vi "UHR-Fleezers Control (host) - 12.2.vi"() -> ()   [LabVIEW 2014] (continued)
        n1769 = local write "Saved Stage Positions"(w2524) -> ()
      }
      event "Move to Position": Value Change {
        n1770 = event-data() -> ()  [unwired: 1 in, 5 out]
        n1771 = flat-sequence {
          tunnel: w2531 -> [w2540]
          tunnel: w2530 -> [w2539]
          tunnel: [w2533] -> w2529
          tunnel: w2529 -> [w2550]
          frame #0 {
            # "Only change move time when saving move is T and calibrating is F"
            n1772 = local read "Saved Stage Positions"() -> (w2541:dbl[][])
            n1773 = property on="Saving Move" class="Bool (strict)"() -> ("Value"=w2534:bool)  [unwired: 2 in, 2 out]
            n1774 = property on="Calibrating..." class="Bool (strict)"() -> ("Value"=w2537:bool)  [unwired: 2 in, 2 out]
            n1775 = local read "Position"() -> (w2533:dbl)
            n1776 = call <vilib>:"Beep.vi"() -> ()  [unwired: 3 in, 9 out]
            n1777 = Not(x=w2537) -> (.not. x?=w2535:bool)
            n1778 = And(x=w2534, y=w2535) -> (x .and. y?=w2536:bool)
            n1779 = local write "Stage Moving"(TRUE ("Stage Moving")) -> ()
            n1780 = case shown="True" w2536 {
              frame False {
              }
              frame True {
                n1781 = Get Date/Time In Seconds() -> (seconds since 1Jan1904=w2549:timestamp)
                n1782 = Format Date/Time String(time format string (%c)="%H:%M:%S%3u", seconds (now)=w2549, UTC format=TRUE) -> (date/time string=w2546:string)
                n1783 = call <vilib>:"Space Constant.vi"() -> ("String"=w2545:string)
                n1784 = Concatenate Strings(w2546, w2545, "moving") -> (w2543:string)
                n1785 = property on="Move Time" class="Str"("Val(Sgnl)"=w2543) -> ()  [unwired: 2 in, 2 out]
              }
            }
            n1786 = call "move to saved stage position.vi"("error in"=w2539, "Stage VISA resource name in"=w2540, "Position"=w2533, "Saved Stage Positions"=w2541) -> ("error out"=w2538:errorcluster)  [unwired: 1 out]
            n1787 = local write "Stage Control Serial Error"(w2538) -> ()
          }
          frame #1 {
            n1788 = call <vilib>:"Beep.vi"() -> ()  [unwired: 3 in, 9 out]
            n1789 = property on="Saving Move" class="Bool (strict)"() -> ("Value"=w2554:bool)  [unwired: 2 in, 2 out]
            n1790 = local write "Stage Moving"(FALSE ("Stage Moving")) -> ()
            n1791 = property on="Calibrating..." class="Bool (strict)"() -> ("Value"=w2551:bool)  [unwired: 2 in, 2 out]
            n1792 = Not(x=w2551) -> (.not. x?=w2553:bool)
            n1793 = And(x=w2554, y=w2553) -> (x .and. y?=w2552:bool)
            n1794 = case shown="True" w2552 {
              tunnel: w2550 -> [_ w2556]
              frame False {
              }
              frame True {
                n1795 = Get Date/Time In Seconds() -> (seconds since 1Jan1904=w2564:timestamp)
                n1796 = Format Date/Time String(time format string (%c)="%H:%M:%S%3u", seconds (now)=w2564, UTC format=TRUE) -> (date/time string=w2561:string)
                n1797 = Number To Decimal String(number=w2556, width (-)=1) -> (decimal integer string=w2557:string)
                n1798 = call <vilib>:"Space Constant.vi"() -> ("String"=w2560:string)
                n1799 = Concatenate Strings(w2561, w2560, w2557) -> (w2559:string)
                n1800 = property on="Move Time" class="Str"("Val(Sgnl)"=w2559) -> ()  [unwired: 2 in, 2 out]
              }
            }
          }
        }
      }
      event "Move Cap. 1 (DNA Bottom)": Value Change {
        n1801 = event-data() -> ()  [unwired: 1 in, 5 out]
        n1802 = local write "Move Cap. 1 (DNA Bottom)"(FALSE ("Move Cap. 1 (DNA Right)")) -> ()
        n1803 = flat-sequence {
          tunnel: w2568 -> [w2571]
          tunnel: w2569 -> [w2572]
          tunnel: [w2572] -> w2566
          tunnel: [w2571] -> w2565
          tunnel: w2566 -> [w2574]
          tunnel: w2565 -> [w2573]
          frame #0 {
            n1804 = property on="Sample Channel\nFlow" class="Bool (strict)"("Val(Sgnl)"="Cap 1 Samp Flow ON") -> ()  [unwired: 2 in, 2 out]
          }
          frame #1 {
            n1805 = local read "Saved Stage Positions"() -> (w2584:dbl[][])
            n1806 = local write "Stage Moving"(TRUE ("Stage Moving")) -> ()
            n1807 = Array Subset(array=w2584, index (row)=0 ("index"), length (row)=1 ("length"), index (col)=1 ("index"), length (col)=3 ("length")) -> (w2581:dbl[][])
            n1808 = Reshape Array(w2581, 3 ("dimension size")) -> (w2579:dbl[])
            n1809 = Array To Cluster(array=w2579) -> (cluster=w2578:cluster{"[0]":dbl, "[1]":dbl, "[2]":dbl})
            n1810 = call "Set Stage Position.vi"("Position"=w2578, "error in"=w2573, "VISA resource name in"=w2574) -> ("error out"=w2577:errorcluster)  [unwired: 2 out]
            n1811 = local write "Stage Control Serial Error"(w2577) -> ()
          }
          frame #2 {
            n1812 = local write "Stage Moving"(FALSE ("Stage Moving")) -> ()
            n1813 = case shown="True" "Cap 1 Flow ON" {
              frame False {
              }
              frame True {
                n1814 = property on="Inject Pump 1" class="Bool (strict)"("Val(Sgnl)"=TRUE ("Value (Signaling)")) -> ()  [unwired: 2 in, 2 out]
              }
            }
            n1815 = call <vilib>:"Beep.vi"() -> ()  [unwired: 3 in, 9 out]
          }
          frame #3 {
            n1816 = property on="Sample Channel\nFlow" class="Bool (strict)"("Val(Sgnl)"=FALSE ("Value (Signaling)")) -> ()  [unwired: 2 in, 2 out]
            n1817 = local read "Cap. 2 BD T1?\n(ADig T1, DNA T2)"() -> (w2591:bool)
            n1818 = case shown="True" w2591 {
              tunnel: "Cap 1 T ON" -> [w2593 w2594]
              frame False {
                n1819 = property on="Trap 1 (ON/OFF)" class="Bool (strict)"("Val(Sgnl)"=w2593) -> ()  [unwired: 2 in, 2 out]
              }
              frame True {
                n1820 = property on="Trap 2 (ON/OFF)" class="Bool (strict)"("Val(Sgnl)"=w2594) -> ()  [unwired: 2 in, 2 out]
              }
            }
            n1821 = property on="Got DNA bead" class="Bool (strict)"("Key Focus"=TRUE) -> ()  [unwired: 2 in, 2 out]
          }
        }
      }
      event "Move Cap. 2 (ADig Top)": Value Change {
        n1822 = event-data() -> ()  [unwired: 1 in, 5 out]
        n1823 = local write "Move Cap. 2 (ADig Top)"(FALSE ("Move Cap. 2 (ADig Left)")) -> ()
        n1824 = flat-sequence {
          tunnel: w2598 -> [w2601]
          tunnel: w2599 -> [w2602]
          tunnel: [w2602] -> w2596
          tunnel: [w2601] -> w2595
          tunnel: w2596 -> [w2604]
          tunnel: w2595 -> [w2603]
          frame #0 {
            n1825 = property on="Sample Channel\nFlow" class="Bool (strict)"("Val(Sgnl)"="Cap 2 Samp Flow ON") -> ()  [unwired: 2 in, 2 out]
          }
          frame #1 {
            n1826 = local read "Saved Stage Positions"() -> (w2614:dbl[][])
            n1827 = local write "Stage Moving"(TRUE ("Stage Moving")) -> ()
            n1828 = Array Subset(array=w2614, index (row)=1 ("index"), length (row)=1 ("length"), index (col)=1 ("index"), length (col)=3 ("length")) -> (w2611:dbl[][])
            n1829 = disable-structure shown="Disabled" {
              frame Disabled {
                w2616 = FALSE ("Value (Signaling)")
                n1830 = property on="Trap 1 (ON/OFF)" class="Bool (strict)"("Val(Sgnl)"=w2616) -> ()  [unwired: 2 in, 2 out]
                n1831 = property on="Trap 1 (ON/OFF)" class="Bool (strict)"("Val(Sgnl)"=w2616) -> ()  [unwired: 2 in, 2 out]
              }
              frame Enabled {
              }
            }
            n1832 = Reshape Array(w2611, 3 ("dimension size")) -> (w2609:dbl[])
            n1833 = Array To Cluster(array=w2609) -> (cluster=w2608:cluster{"[0]":dbl, "[1]":dbl, "[2]":dbl})
            n1834 = call "Set Stage Position.vi"("Position"=w2608, "error in"=w2603, "VISA resource name in"=w2604) -> ("error out"=w2607:errorcluster)  [unwired: 2 out]
            n1835 = local write "Stage Control Serial Error"(w2607) -> ()
          }
          frame #2 {
            n1836 = local write "Stage Moving"(FALSE ("Stage Moving")) -> ()
            n1837 = call <vilib>:"Beep.vi"() -> ()  [unwired: 3 in, 9 out]
            n1838 = case shown="True" "Cap 2 Flow ON" {
              frame False {
              }
              frame True {
                n1839 = property on="Inject Pump 3" class="Bool (strict)"("Val(Sgnl)"=TRUE ("Value (Signaling)")) -> ()  [unwired: 2 in, 2 out]
              }
            }
          }
          frame #3 {
            n1840 = Wait (ms)(milliseconds to wait=u32 500) -> ()  [unwired: 1 out]
          }
          frame #4 {
            n1841 = local read "Cal @ (MHz)"() -> (w2622:dbl)
            n1842 = property on="Sample Channel\nFlow" class="Bool (strict)"("Val(Sgnl)"=FALSE ("Value (Signaling)")) -> ()  [unwired: 2 in, 2 out]
            n1843 = case shown="False" "Cap. 2 BD T1?\n(ADig T1, DNA T2)" {
              tunnel: "Cap 2 T ON" -> [w2627 w2628]
              frame False {
                n1844 = property on="Trap 2 (ON/OFF)" class="Bool (strict)"("Val(Sgnl)"=w2627) -> ()  [unwired: 2 in, 2 out]
              }
              frame True {
                n1845 = property on="Trap 1 (ON/OFF)" class="Bool (strict)"("Val(Sgnl)"=w2628) -> ()  [unwired: 2 in, 2 out]
              }
            }
            n1846 = property on="Got ADig bead" class="Bool (strict)"("Key Focus"=TRUE) -> ()  [unwired: 2 in, 2 out]
            n1847 = local write "Target"("Target\nON?") -> ()
            n1848 = property on="Trap D (MHz)" class="DigNum (strict)"("Val(Sgnl)"=w2622) -> ()  [unwired: 2 in, 2 out]
          }
        }
      }
      event "Read Harvard": Value Change {
        n1849 = event-data() -> ()  [unwired: 1 in, 5 out]
        n1850 = Concatenate Strings("write buffer", "\r") -> (w2633:string)
        n1851 = VISA Write(VISA resource name=w2631, write buffer=w2633, error in (no error)=w2630) -> (VISA resource name out=w2642:refnum<visa-resource-name>, error out=w2641:errorcluster)  [unwired: 1 out]
        n1852 = stacked-sequence {
          tunnel: [w2645] -> w2640
          tunnel: w2642 -> [w2645]
          tunnel: w2641 -> [w2644]
          tunnel: [w2644] -> w2635
          frame #0 {
            n1853 = Wait (ms)(milliseconds to wait=50) -> ()  [unwired: 1 out]
          }
        }
        n1854 = property class="Instr"(reference=w2640, error in=w2635) -> (reference out=w2639:refnum<visa-resource-name>, error out=w2637:errorcluster, "Serial Settings:Number of Bytes at Serial Port"=w2638:u32)
        "Serial Settings:Number of Bytes at Serial Port" <- w2638
        n1855 = VISA Read(VISA resource name=w2639, byte count=w2638, error in (no error)=w2637) -> (read buffer=w2636:string)  [unwired: 3 out]
        "read buffer" <- w2636
        n1856 = Fract/Exp String To Number(string=w2636) -> ()  [unwired: 5 out]
      }
      event "+z", "-z": Value Change {
        n1857 = event-data() -> ()  [unwired: 1 in, 5 out]
        n1858 = flat-sequence {
          tunnel: w2646 -> [w2668]
          tunnel: w2647 -> [w2648]
          frame #0 {
            n1859 = call "Read Stage Position.vi"("error in"=w2668, "VISA resource name in"=w2648) -> ("Current Position"=w2653:cluster{dbl, dbl, dbl}, "error out"=w2666:errorcluster, "VISA resource name out"=w2667:refnum<visa-resource-name>)  [unwired: 1 out]
            n1860 = local read "Saved Stage Positions"() -> (w2677:dbl[][])
            n1861 = Divide(x="z nudge increment (um)", y=1000.0) -> (x/y=w2665:dbl)
            n1862 = Boolean To (0,1)(Boolean="+z") -> (0, 1=w2657:i16)
            n1863 = Boolean To (0,1)(Boolean="-z") -> (0, 1=w2658:i16)
            n1864 = Array Subset(array=w2677, index (row)=1 ("index"), length (row)=1 ("length"), index (col)=1 ("index"), length (col)=3 ("length")) -> (w2674:dbl[][])
            n1865 = Multiply(x=w2657, y=w2665) -> (x*y=w2661:dbl)
            n1866 = Multiply(x=w2658, y=w2665) -> (x*y=w2659:dbl)
            n1867 = Unbundle(w2653) -> (w2651:dbl, w2650:dbl, w2654:dbl)
            n1868 = Negate(x=w2659) -> (-x=w2660:dbl)
            n1869 = Reshape Array(w2674, 3 ("dimension size")) -> (w2672:dbl[])
            n1870 = Add(x=w2661, y=w2660) -> (x+y=w2662:dbl)
            n1871 = Array To Cluster(array=w2672) -> ()  [unwired: 1 out]
            n1872 = Add(x=w2662, y=w2654) -> (x+y=w2652:dbl)
            n1873 = Bundle(cluster=w2653, w2651, w2650, w2652) -> (w2649:cluster{dbl, dbl, dbl})
            n1874 = call "Set Stage Position.vi"("Position"=w2649, "error in"=w2666, "VISA resource name in"=w2667) -> ("error out"=w2671:errorcluster)  [unwired: 2 out]
            n1875 = local write "Stage Moving"(TRUE ("Stage Moving")) -> ()
            n1876 = local write "Stage Control Serial Error"(w2671) -> ()
          }
          frame #1 {
            n1877 = local write "Stage Moving"(FALSE ("Stage Moving")) -> ()
            n1878 = call <vilib>:"Beep.vi"() -> ()  [unwired: 3 in, 9 out]
          }
        }
      }
      event "Cal/Data Acq. Spot": Value Change {
        n1879 = event-data() -> ()  [unwired: 1 in, 5 out]
        n1880 = flat-sequence {
          tunnel: w2686 -> [w2690]
          tunnel: w2687 -> [w2691]
          tunnel: [w2691] -> w2683
          tunnel: [w2690] -> w2682
          tunnel: w2683 -> [w2696]
          tunnel: w2682 -> [w2695]
          tunnel: ["Cal @ (MHz)"] -> w2680
          tunnel: [w2700] -> w2684
          tunnel: w2680 -> [w2700]
          tunnel: w2684 -> [w2711]
          tunnel: ["W/ Offset 1"] -> w2681
          tunnel: w2684 -> [w2732]
          tunnel: w2681 -> [w2730]
          frame #0 {
            n1881 = property on="Sample Channel\nFlow" class="Bool (strict)"("Val(Sgnl)"="Daq spot flow on") -> ()  [unwired: 2 in, 2 out]
            n1882 = Wait (ms)(milliseconds to wait=u32 250) -> ()  [unwired: 1 out]
          }
          frame #1 {
            n1883 = local read "Saved Stage Positions"() -> (w2693:dbl[][])
            n1884 = property on="Trap D (MHz)" class="DigNum (strict)"("Val(Sgnl)"="Cal @ (MHz)") -> ()  [unwired: 2 in, 2 out]
            n1885 = local write "Stage Moving"(TRUE ("Stage Moving")) -> ()
            n1886 = call "move to saved stage position.vi"("error in"=w2695, "Stage VISA resource name in"=w2696, "Position"="Cal Stage Position", "Saved Stage Positions"=w2693) -> ("error out"=w2694:errorcluster)  [unwired: 1 out]
            n1887 = local write "Stage Control Serial Error"(w2694) -> ()
          }
          frame #2 {
            n1888 = local write "Stage Moving"(FALSE ("Stage Moving")) -> ()
            n1889 = property on="Sample Channel\nFlow" class="Bool (strict)"("Val(Sgnl)"="Flow ON\nduring cal?") -> ()  [unwired: 2 in, 2 out]
            n1890 = call <vilib>:"Beep.vi"() -> ()  [unwired: 3 in, 9 out]
          }
          frame #3 {
            n1891 = local read "Wait Before Save (s)"() -> (w2703:u32)
            n1892 = Multiply(x=w2703, y=u32 1000 ("milliseconds to wait")) -> (x*y=w2704:u32)
            n1893 = Wait (ms)(milliseconds to wait=w2704) -> ()  [unwired: 1 out]
          }
          frame #4 {
            n1894 = property on="Save Calibration" class="Bool (strict)"("Val(Sgnl)"=TRUE ("Value (Signaling)")) -> ()  [unwired: 2 in, 2 out]
          }
          frame #5 {
            n1895 = Wait (ms)(milliseconds to wait=u32 2000) -> ()  [unwired: 1 out]
          }
          frame #6 {
            # "Check to see if \nsaving done"
            n1896 = while {
              stop <- w2707 stop-if-true
              n1897 = local read "Saving..."() -> (w2708:bool)
              n1898 = Wait (ms)(milliseconds to wait=u32 100) -> ()  [unwired: 1 out]
              n1899 = Not(x=w2708) -> (.not. x?=w2707:bool)
            }
          }
          frame #7 {
            n1900 = case shown="True" "W/ Offset 1" {
              tunnel: w2711 -> [_ w2712]
              frame False {
              }
              frame True {
                n1901 = stacked-sequence {
                  tunnel: w2712 -> [_ _ _ _ _ _ _ w2729]
                  frame #0 {
                    n1902 = property on="Trap D (MHz)" class="DigNum (strict)"("Val(Sgnl)"="Offset 1 Start (MHz)") -> ()  [unwired: 2 in, 2 out]
                    n1903 = Replace Array Subset(array=u32[] [0] ("Index Values"), new element="Offset 1 Set", index=0) -> (w2713:u32[])
                    n1904 = property on="Saved AOD Raster Scan Parameter Sets" class="Arr (strict)"("Index Values"=w2713) -> ()  [unwired: 2 in, 2 out]
                  }
                  frame #1 {
                    n1905 = Wait (ms)(milliseconds to wait=u32 200) -> ()  [unwired: 1 out]
                  }
                  frame #2 {
                    n1906 = property on="Load parameters" class="Bool (strict)"("Val(Sgnl)"=TRUE ("Value (Signaling)")) -> ()  [unwired: 2 in, 2 out]
                  }
                  frame #3 {
                    n1907 = Wait (ms)(milliseconds to wait=u32 200) -> ()  [unwired: 1 out]
                  }
                  frame #4 {
                    n1908 = property on="Trap Raster Scan" class="Bool (strict)"("Val(Sgnl)"=TRUE ("Value (Signaling)")) -> ()  [unwired: 2 in, 2 out]
                  }
                  frame #5 {
                    n1909 = Wait (ms)(milliseconds to wait=u32 2000) -> ()  [unwired: 1 out]
                  }
                  frame #6 {
                    n1910 = while {
                      stop <- w2726 stop-if-true
                      n1911 = local read "Raster Scanning..."() -> (w2728:bool)
                      n1912 = local read "Saving..."() -> (w2724:bool)
                      n1913 = Wait (ms)(milliseconds to wait=u32 100) -> ()  [unwired: 1 out]
                      n1914 = Not(x=w2724) -> (.not. x?=w2723:bool)
                      n1915 = Not(x=w2728) -> (.not. x?=w2725:bool)
                      n1916 = And(x=w2725, y=w2723) -> (x .and. y?=w2726:bool)
                    }
                  }
                  frame #7 {
                    n1917 = property on="Trap D (MHz)" class="DigNum (strict)"("Val(Sgnl)"=w2729) -> ()  [unwired: 2 in, 2 out]
                  }
                }
              }
            }
          }
          frame #8 {
            n1918 = local read "Save ave N"() -> (w2731:dbl)
            n1919 = case shown="False" "W/ Offset 2" {
              tunnel: w2732 -> [_ w2739]
              tunnel: w2731 -> [_ w2738]
              tunnel: w2730 -> [w2734 _]
              frame False {
                n1920 = case shown="False" w2734 {
                  frame False {
                    n1921 = Multiply(x="Cal read wait (s)", y=u32 1000 ("milliseconds to wait")) -> (x*y=w2736:u32)
                    n1922 = Wait (ms)(milliseconds to wait=w2736) -> ()  [unwired: 1 out]
                  }
                  frame True {
                  }
                }
              }
              frame True {
                n1923 = stacked-sequence {
                  tunnel: w2739 -> [_ _ _ _ _ _ _ _ _ w2760 _ _]
                  tunnel: w2738 -> [_ _ _ _ _ _ _ _ _ w2758 _ _]
                  frame #0 {
                    n1924 = property on="Save ave N" class="DigNum (strict)"("Val(Sgnl)"=1.0 ("Value (Signaling)")) -> ()  [unwired: 2 in, 2 out]
                  }
                  frame #1 {
                    n1925 = Wait (ms)(milliseconds to wait=u32 500) -> ()  [unwired: 1 out]
                  }
                  frame #2 {
                    n1926 = property on="Trap D (MHz)" class="DigNum (strict)"("Val(Sgnl)"="Offset 2 Start (MHz)") -> ()  [unwired: 2 in, 2 out]
                    n1927 = Replace Array Subset(array=u32[] [0] ("Index Values"), new element="Offset 2 Set", index=0) -> (w2744:u32[])
                    n1928 = property on="Saved AOD Raster Scan Parameter Sets" class="Arr (strict)"("Index Values"=w2744) -> ()  [unwired: 2 in, 2 out]
                  }
                  frame #3 {
                    n1929 = Wait (ms)(milliseconds to wait=u32 500) -> ()  [unwired: 1 out]
                  }
                  frame #4 {
                    n1930 = property on="Load parameters" class="Bool (strict)"("Val(Sgnl)"=TRUE ("Value (Signaling)")) -> ()  [unwired: 2 in, 2 out]
                  }
                  frame #5 {
                    n1931 = Wait (ms)(milliseconds to wait=u32 500) -> ()  [unwired: 1 out]
                  }
                  frame #6 {
                    n1932 = property on="Trap Raster Scan" class="Bool (strict)"("Val(Sgnl)"=TRUE ("Value (Signaling)")) -> ()  [unwired: 2 in, 2 out]
                  }
                  frame #7 {
                    n1933 = Wait (ms)(milliseconds to wait=u32 2000) -> ()  [unwired: 1 out]
                  }
                  frame #8 {
                    n1934 = while {
                      stop <- w2753 stop-if-true
                      n1935 = local read "Raster Scanning..."() -> (w2756:bool)
                      n1936 = local read "Saving..."() -> (w2754:bool)
                      n1937 = Wait (ms)(milliseconds to wait=u32 100) -> ()  [unwired: 1 out]
                      n1938 = Not(x=w2754) -> (.not. x?=w2752:bool)
                      n1939 = Not(x=w2756) -> (.not. x?=w2755:bool)
                      n1940 = And(x=w2755, y=w2752) -> (x .and. y?=w2753:bool)
                    }
                  }
                  frame #9 {
                    n1941 = property on="Trap D (MHz)" class="DigNum (strict)"("Val(Sgnl)"=w2760) -> ()  [unwired: 2 in, 2 out]
                    n1942 = property on="Saved AOD Raster Scan Parameter Sets" class="Arr (strict)"("Index Values"=u32[] [0]) -> ()  [unwired: 2 in, 2 out]
                    n1943 = property on="Save ave N" class="DigNum (strict)"("Val(Sgnl)"=w2758) -> ()  [unwired: 2 in, 2 out]
                  }
                  frame #10 {
                    n1944 = Wait (ms)(milliseconds to wait=u32 500) -> ()  [unwired: 1 out]
                  }
                  frame #11 {
                    n1945 = property on="Load parameters" class="Bool (strict)"("Val(Sgnl)"=TRUE ("Value (Signaling)")) -> ()  [unwired: 2 in, 2 out]
                  }
                }
              }
            }
          }
          frame #9 {
            n1946 = property on="Read Cal" class="Bool (strict)"("Val(Sgnl)"=TRUE ("Value (Signaling)")) -> ()  [unwired: 2 in, 2 out]
          }
          frame #10 {
            n1947 = Wait (ms)(milliseconds to wait=u32 1000) -> ()  [unwired: 1 out]
          }
          frame #11 {
            n1948 = property on="Fish" class="Bool (strict)"("Val(Sgnl)"=TRUE ("Value (Signaling)")) -> ()  [unwired: 2 in, 2 out]
          }
        }
        n1949 = local write "Cal/Data Acq. Spot"(FALSE ("Cal/Data Acq. Spot")) -> ()
      }
      event "Dump Beads": Value Change {
        n1950 = event-data() -> ()  [unwired: 1 in, 5 out]
        n1951 = flat-sequence {
          tunnel: ["Dump spot flow on?"] -> w2766
          tunnel: [w2778] -> w2767
          tunnel: w2766 -> [w2778]
          tunnel: w2770 -> [w2783]
          tunnel: w2769 -> [w2782]
          tunnel: [w2780] -> w2768
          tunnel: w2767 -> [w2780]
          tunnel: w2768 -> [w2794]
          frame #0 {
            w2771 = FALSE ("Value (Signaling)")
            n1952 = local read "Saving..."() -> (w2773:bool)
            n1953 = local write "Dump Beads"(FALSE ("Dump Beads")) -> ()
            n1954 = property on="Inject Pump 3" class="Bool (strict)"("Val(Sgnl)"=w2771) -> ()  [unwired: 2 in, 2 out]
            n1955 = property on="Inject Pump 1" class="Bool (strict)"("Val(Sgnl)"=w2771) -> ()  [unwired: 2 in, 2 out]
            n1956 = local write "Stop Saving"(w2773) -> ()
            n1957 = local write "Fish"(w2771) -> ()
          }
          frame #1 {
            w2774 = TRUE
            w2775 = FALSE ("Fl. Triggered...")
            n1958 = case shown="True" "Dump spot flow on?" {
              frame False {
              }
              frame True {
                n1959 = property on="Sample Channel\nFlow" class="Bool (strict)"("Val(Sgnl)"=TRUE ("Stage Moving")) -> ()  [unwired: 2 in, 2 out]
              }
            }
            n1960 = local write "Fl. Triggered..."(w2775) -> ()
            n1961 = local write "Tether"(w2775) -> ()
            n1962 = local write "Multiple tether"(w2775) -> ()
            n1963 = local write "Good tether"(w2775) -> ()
            n1964 = property on="Green ON/Interlacing" class="Bool (strict)"("Val(Sgnl)"=w2775) -> ()  [unwired: 2 in, 2 out]
            n1965 = property on="Trap Pos. FB ON" class="Bool (strict)"("Val(Sgnl)"=w2775) -> ()  [unwired: 2 in, 2 out]
            n1966 = property on="Trap Trig. Fl." class="Bool (strict)"("Val(Sgnl)"=w2775) -> ()  [unwired: 2 in, 2 out]
            n1967 = local write "Bad fit"(w2775) -> ()
            n1968 = local write "Hysteresis"(w2775) -> ()
            n1969 = property on="Fl. Triggered..." class="Bool (strict)"("Val(Sgnl)"=w2775) -> ()  [unwired: 2 in, 2 out]
            n1970 = local write "Restart DMA? (AOD)"(w2774) -> ()
            n1971 = local write "Save scans"(w2774) -> ()
            n1972 = property on="Dip for Protein" class="Bool (strict)"("Val(Sgnl)"=w2775) -> ()  [unwired: 2 in, 2 out]
            n1973 = property on="Pause dwell" class="Bool (strict)"("Val(Sgnl)"=w2775) -> ()  [unwired: 2 in, 2 out]
          }
          frame #2 {
            n1974 = property on="Trap Pos. FB Offset Factor" class="DigNum (strict)"("Val(Sgnl)"=i64 0 ("Value (Signaling)")) -> ()  [unwired: 2 in, 2 out]
          }
          frame #3 {
            n1975 = local read "Saved Stage Positions"() -> (w2784:dbl[][])
            n1976 = Array Subset(array=w2784, index (row)=3 ("index"), length (row)=1 ("length"), index (col)=1 ("index"), length (col)=3 ("length")) -> (w2789:dbl[][])
            n1977 = local write "Stage Moving"(TRUE ("Stage Moving")) -> ()
            n1978 = Reshape Array(w2789, 3 ("dimension size")) -> (w2787:dbl[])
            n1979 = Array To Cluster(array=w2787) -> (cluster=w2786:cluster{"[0]":dbl, "[1]":dbl, "[2]":dbl})
            n1980 = call "Set Stage Position.vi"("Position"=w2786, "error in"=w2782, "VISA resource name in"=w2783) -> ()  [unwired: 3 out]
          }
          frame #4 {
            w2795 = FALSE ("Value (Signaling)")
            n1981 = case shown="True" w2794 {
              frame False {
              }
              frame True {
                n1982 = property on="Sample Channel\nFlow" class="Bool (strict)"("Val(Sgnl)"=FALSE ("Stage Moving")) -> ()  [unwired: 2 in, 2 out]
              }
            }
            n1983 = property on="Trap 1 (ON/OFF)" class="Bool (strict)"("Val(Sgnl)"=w2795) -> ()  [unwired: 2 in, 2 out]
            n1984 = property on="Trap 2 (ON/OFF)" class="Bool (strict)"("Val(Sgnl)"=w2795) -> ()  [unwired: 2 in, 2 out]
            n1985 = call <vilib>:"Beep.vi"() -> ()  [unwired: 3 in, 9 out]
            n1986 = local write "Fish"(FALSE ("Fish for Tether")) -> ()
          }
          frame #5 {
            n1987 = property on="Move Cap. 2 (ADig Top)" class="Bool (strict)"("Val(Sgnl)"=TRUE ("Value (Signaling)")) -> ()  [unwired: 2 in, 2 out]
            n1988 = property on="Tab Control" class="TabCtl (strict)"("Val(Sgnl)"=T34."Status" ("Value (Signaling)")) -> ()  [unwired: 2 in, 2 out]
          }
        }
      }
      event "Dip for Protein": Value Change {
        n1989 = event-data() -> ()  [unwired: 1 in, 5 out]
        n1990 = local read "Calibrating..."() -> (w2802:bool)
        n1991 = local read "Saving Move"() -> (w2800:bool)
        n1992 = Not(x=w2802) -> (.not. x?=w2801:bool)
        n1993 = And(x=w2800, y=w2801) -> (x .and. y?=w2799:bool)
        n1994 = case shown="True" "Dip for Protein" {
          tunnel: w2805 -> [_ w2808]
          tunnel: w2804 -> [_ w2807]
          tunnel: w2799 -> [_ w2806]
          frame False {
          }
          frame True {
            n1995 = while {
              tunnel: w2808 -> [w2821]
              tunnel: w2807 -> [w2820]
              tunnel: w2806 -> [w2809]
              i -> [w2816]
              stop <- w2811 stop-if-true
              n1996 = Increment(x=w2816) -> (x+1=→"Dip #":i32)
              n1997 = flat-sequence {
                tunnel: w2820 -> [w2832]
                tunnel: w2821 -> [w2833]
                tunnel: [w2833] -> w2825
                tunnel: [w2832] -> w2824
                tunnel: [w2826] -> w2812
                tunnel: [w2840] -> w2819
                tunnel: [w2841] -> w2818
                tunnel: w2825 -> [w2842]
                tunnel: w2824 -> [w2843]
                tunnel: [w2838] -> w2813
                tunnel: w2812 -> [w2838]
                tunnel: w2809 -> [w2837]
                tunnel: ["Dip Stage \nPosition"] -> w2810
                tunnel: [w2860] -> w2823
                tunnel: w2819 -> [w2860]
                tunnel: [w2859] -> w2822
                tunnel: w2818 -> [w2859]
                tunnel: [w2856] -> w2817
                tunnel: [w2855] -> w2814
                tunnel: w2813 -> [w2855]
                tunnel: w2809 -> [w2854]
                tunnel: w2810 -> [w2853]
                tunnel: w2822 -> [w2892]
                tunnel: w2823 -> [w2893]
                tunnel: w2817 -> [w2894]
                tunnel: w2814 -> [w2891]
                tunnel: w2809 -> [w2890]
                tunnel: w2809 -> [w2889]
                tunnel: [w2977] -> w2811
                frame #0 {
                  n1998 = local read "Trap Pos. FB ON"() -> (w2826:bool)
                  n1999 = Compound Arithmetic op=AND("Flow ON\nduring dip?", "FB OFF when \nflow ON", w2826) -> (w2827:bool)
                  n2000 = case shown="True" "Move trap \nbefore dip move?" {
                    frame False {
                    }
                    frame True {
                      n2001 = property on="Trap D (MHz)" class="DigNum (strict)"("Val(Sgnl)"="Dipping D (MHz)") -> ()  [unwired: 2 in, 2 out]
                    }
                  }
                  n2002 = property on="Green ON/Interlacing" class="Bool (strict)"("Val(Sgnl)"="Green ON\nbefore dip?") -> ()  [unwired: 2 in, 2 out]
                  n2003 = property on="Sample Channel\nFlow" class="Bool (strict)"("Val(Sgnl)"="Flow ON\nduring dip?") -> ()  [unwired: 2 in, 2 out]
                  n2004 = case shown="True" w2827 {
                    frame False {
                    }
                    frame True {
                      n2005 = property on="Trap Pos. FB ON" class="Bool (strict)"("Val(Sgnl)"=FALSE ("Value (Signaling)")) -> ()  [unwired: 2 in, 2 out]
                    }
                  }
                }
                frame #1 {
                  n2006 = local read "Saved Stage Positions"() -> (w2844:dbl[][])
                  n2007 = local write "Cancel dwell"(FALSE ("Cancel dwell")) -> ()
                  n2008 = call "move to saved stage position.vi"("error in"=w2843, "Stage VISA resource name in"=w2842, "Position"="Dip Stage \nPosition", "Saved Stage Positions"=w2844) -> ("VISA resource name out"=w2840:refnum<visa-resource-name>, "error out"=w2841:errorcluster)
                  n2009 = case shown="True" w2837 {
                    frame False {
                    }
                    frame True {
                      n2010 = Get Date/Time In Seconds() -> (seconds since 1Jan1904=w2851:timestamp)
                      n2011 = call <vilib>:"Space Constant.vi"() -> ("String"=w2848:string)
                      n2012 = local write "Stage Moving"(TRUE) -> ()
                      n2013 = Format Date/Time String(time format string (%c)="%H:%M:%S%3u", seconds (now)=w2851, UTC format=TRUE) -> (date/time string=w2849:string)
                      n2014 = Concatenate Strings(w2849, w2848, "moving") -> (w2846:string)
                      n2015 = property on="Move Time" class="Str"("Val(Sgnl)"=w2846) -> ()  [unwired: 2 in, 2 out]
                    }
                  }
                }
                frame #2 {
                  n2016 = node-c288() -> (w2858:T26)  [unwired: 4 in]
                  n2017 = timed-loop {
                    timing: w2858 -> [_]
                    timing-out: [_] -> w2857
                    tunnel: [w2874] -> w2856
                    i -> [w2871]
                    stop <- w2875 stop-if-true
                    n2018 = node-c288() -> ()  [unwired: 1 in, 1 out]
                    n2019 = Greater Or Equal?(x=w2871, y="Dip Duration (s)") -> (x >= y?=w2883:bool)
                    n2020 = local read "Dip for Protein"() -> (w2876:bool)
                    n2021 = local read "Dump Beads"() -> (w2873:bool)
                    n2022 = local read "Cancel dwell"() -> (w2882:bool)
                    n2023 = local read "Pause dwell"() -> (w2879:bool)
                    n2024 = Not(x=w2876) -> (.not. x?=w2881:bool)
                    n2025 = Compound Arithmetic op=OR(w2882, w2883, w2881) -> (w2880:bool)
                    n2026 = Select(t=FALSE, s=w2879, f=w2880) -> (s? t:f=w2877:bool)
                    n2027 = Not(x=w2873) -> (.not. x?=w2872:bool)
                    n2028 = node-c288() -> ()  [unwired: 1 in, 1 out]
                    n2029 = And(x=w2876, y=w2872) -> (x .and. y?=w2874:bool)
                    n2030 = Or(x=w2877, y=w2873) -> (x .or. y?=w2875:bool)
                    "Dip Time (s)" <- w2871
                  }
                  n2031 = case shown="True" w2854 {
                    tunnel: w2853 -> [_ w2861]
                    frame False {
                    }
                    frame True {
                      n2032 = Get Date/Time In Seconds() -> (seconds since 1Jan1904=w2869:timestamp)
                      n2033 = call <vilib>:"Space Constant.vi"() -> ("String"=w2866:string)
                      n2034 = Number To Decimal String(number=w2861, width (-)=1) -> (decimal integer string=w2864:string)
                      n2035 = local write "Stage Moving"(FALSE) -> ()
                      n2036 = Format Date/Time String(time format string (%c)="%H:%M:%S%3u", seconds (now)=w2869, UTC format=TRUE) -> (date/time string=w2867:string)
                      n2037 = Concatenate Strings(w2867, w2866, w2864) -> (w2865:string)
                      n2038 = property on="Move Time" class="Str"("Val(Sgnl)"=w2865) -> ()  [unwired: 2 in, 2 out]
                    }
                  }
                  n2039 = node-c288(w2857) -> ()  [unwired: 1 out]
                }
                frame #3 {
                  n2040 = case shown="True" w2894 {
                    tunnel: w2893 -> [_ w2902]
                    tunnel: w2892 -> [_ w2901]
                    tunnel: w2891 -> [_ w2898]
                    tunnel: w2890 -> [_ w2897]
                    tunnel: w2889 -> [_ w2895]
                    frame False {
                    }
                    frame True {
                      n2041 = flat-sequence {
                        tunnel: w2901 -> [w2906]
                        tunnel: w2902 -> [w2907]
                        tunnel: [w2907] -> w2900
                        tunnel: [w2906] -> w2899
                        tunnel: w2898 -> [w2903]
                        tunnel: w2900 -> [w2919]
                        tunnel: w2899 -> [w2918]
                        tunnel: w2897 -> [w2915]
                        tunnel: ["Return Stage \nPosition"] -> w2896
                        tunnel: w2898 -> [w2937]
                        tunnel: w2896 -> [w2935]
                        tunnel: w2895 -> [w2934]
                        frame #0 {
                          n2042 = local read "Sample Channel\nFlow"() -> (w2905:bool)
                          n2043 = case shown="True" w2905 {
                            tunnel: "Flow ON \nduring return\nfrom dip?" -> [w2908 w2911]
                            tunnel: w2903 -> [_ w2910]
                            frame False {
                              n2044 = case shown="True" w2908 {
                                frame False {
                                }
                                frame True {
                                n2045 = property on="Sample Channel\nFlow" class="Bool (strict)"("Val(Sgnl)"=TRUE ("Value (Signaling)")) -> ()  [unwired: 2 in, 2 out]
                                }
                              }
                            }
                            frame True {
                              n2046 = case shown="False" w2911 {
                                tunnel: w2910 -> [w2912 _]
                                frame False {
                                n2047 = property on="Trap Pos. FB ON" class="Bool (strict)"("Val(Sgnl)"=w2912) -> ()  [unwired: 2 in, 2 out]
                                n2048 = property on="Sample Channel\nFlow" class="Bool (strict)"("Val(Sgnl)"=FALSE ("Value (Signaling)")) -> ()  [unwired: 2 in, 2 out]
                                }
                                frame True {
                                }
                              }
                            }
                          }
                        }
                        frame #1 {
                          # "For turning on green laser before stage reaches lower spot"
                          n2049 = case shown="True" "Green ON\nafter start\nreturn?" {
                            frame False {
                            }
                            frame True {
                              n2050 = flat-sequence {
                                frame #0 {
                                n2051 = Multiply(x="Green delay after \nstart return (s)", y=1000.0) -> (x*y=w2931:dbl)
                                n2052 = Wait (ms)(milliseconds to wait=w2931) -> ()  [unwired: 1 out]
                                }
                                frame #1 {
                                n2053 = property on="Green ON/Interlacing" class="Bool (strict)"("Val(Sgnl)"=TRUE ("Value (Signaling)")) -> ()  [unwired: 2 in, 2 out]
                                }
                              }
                            }
                          }
                          n2054 = local read "Saved Stage Positions"() -> (w2921:dbl[][])
                          n2055 = local write "Cancel dwell"(FALSE ("Cancel dwell")) -> ()
                          n2056 = call "move to saved stage position.vi"("error in"=w2918, "Stage VISA resource name in"=w2919, "Position"="Return Stage \nPosition", "Saved Stage Positions"=w2921) -> ("error out"=w2920:errorcluster)  [unwired: 1 out]
                          n2057 = local write "Stage Control Serial Error"(w2920) -> ()
                          n2058 = case shown="True" w2915 {
                            frame False {
                            }
                            frame True {
                              n2059 = Get Date/Time In Seconds() -> (seconds since 1Jan1904=w2928:timestamp)
                              n2060 = call <vilib>:"Space Constant.vi"() -> ("String"=w2925:string)
                              n2061 = local write "Stage Moving"(TRUE) -> ()
                              n2062 = Format Date/Time String(time format string (%c)="%H:%M:%S%3u", seconds (now)=w2928, UTC format=TRUE) -> (date/time string=w2926:string)
                              n2063 = Concatenate Strings(w2926, w2925, "moving") -> (w2923:string)
                              n2064 = property on="Move Time" class="Str"("Val(Sgnl)"=w2923) -> ()  [unwired: 2 in, 2 out]
                            }
                          }
                        }
                        frame #2 {
                          n2065 = case shown="True" w2934 {
                            tunnel: w2935 -> [_ w2941]
                            frame False {
                            }
                            frame True {
                              n2066 = Get Date/Time In Seconds() -> (seconds since 1Jan1904=w2949:timestamp)
                              n2067 = call <vilib>:"Space Constant.vi"() -> ("String"=w2946:string)
                              n2068 = Number To Decimal String(number=w2941, width (-)=1) -> (decimal integer string=w2944:string)
                              n2069 = local write "Stage Moving"(FALSE) -> ()
                              n2070 = Format Date/Time String(time format string (%c)="%H:%M:%S%3u", seconds (now)=w2949, UTC format=TRUE) -> (date/time string=w2947:string)
                              n2071 = Concatenate Strings(w2947, w2946, w2944) -> (w2945:string)
                              n2072 = property on="Move Time" class="Str"("Val(Sgnl)"=w2945) -> ()  [unwired: 2 in, 2 out]
                            }
                          }
                          n2073 = case shown="True" "Move trap after return?" {
                            frame False {
                            }
                            frame True {
                              n2074 = property on="Trap D (MHz)" class="DigNum (strict)"("Val(Sgnl)"="Dip Trap D 2 (MHz)") -> ()  [unwired: 2 in, 2 out]
                            }
                          }
                          n2075 = property on="Trap Pos. FB ON" class="Bool (strict)"("Val(Sgnl)"=w2937) -> ()  [unwired: 2 in, 2 out]
                          n2076 = case shown="True" "Green ON \nafter return?" {
                            frame False {
                            }
                            frame True {
                              n2077 = property on="Green ON/Interlacing" class="Bool (strict)"("Val(Sgnl)"=TRUE ("Value (Signaling)")) -> ()  [unwired: 2 in, 2 out]
                            }
                          }
                          n2078 = case shown="True" "Save data after return?" {
                            frame False {
                            }
                            frame True {
                              n2079 = property on="Start Saving" class="Bool (strict)"("Val(Sgnl)"=TRUE ("Value (Signaling)")) -> ()  [unwired: 2 in, 2 out]
                            }
                          }
                          n2080 = property on="Sample Channel\nFlow" class="Bool (strict)"("Val(Sgnl)"="Flow ON\nduring daq?") -> ()  [unwired: 2 in, 2 out]
                        }
                        frame #3 {
                          n2081 = node-c288() -> (w2955:T26)  [unwired: 4 in]
                          n2082 = timed-loop {
                            timing: w2955 -> [_]
                            timing-out: [_] -> w2954
                            i -> [w2956]
                            stop <- w2958 stop-if-true
                            n2083 = node-c288() -> ()  [unwired: 1 in, 1 out]
                            n2084 = local read "Dump Beads"() -> (w2957:bool)
                            n2085 = Greater Or Equal?(x=w2956, y="Dwell Duration (s)") -> (x >= y?=w2963:bool)
                            n2086 = local read "Dip for Protein"() -> (w2960:bool)
                            n2087 = Not(x=w2960) -> (.not. x?=w2959:bool)
                            n2088 = Compound Arithmetic op=OR(w2963, "Cancel dwell", w2959) -> (w2962:bool)
                            n2089 = node-c288() -> ()  [unwired: 1 in, 1 out]
                            n2090 = Select(t=FALSE, s="Pause dwell", f=w2962) -> (s? t:f=w2965:bool)
                            n2091 = Or(x=w2965, y=w2957) -> (x .or. y?=w2958:bool)
                            "Dwell Time (s)" <- w2956
                          }
                          n2092 = node-c288(w2954) -> ()  [unwired: 1 out]
                        }
                      }
                    }
                  }
                }
                frame #4 {
                  n2093 = local read "Dip for Protein"() -> (w2974:bool)
                  n2094 = local read "Tether"() -> (w2973:bool)
                  n2095 = local read "Dump Beads"() -> (w2975:bool)
                  n2096 = local write "Cancel dwell"(FALSE ("Cancel dwell")) -> ()
                  n2097 = Not(x=w2973) -> (.not. x?=w2972:bool)
                  n2098 = Not(x=w2974) -> (.not. x?=w2978:bool)
                  n2099 = Not(x="Cont. Repeat Dipping?") -> (.not. x?=w2980:bool)
                  n2100 = Compound Arithmetic op=OR(w2972, w2978, w2980, w2975) -> (w2977:bool)
                }
              }
            }
          }
        }
      }
      event "Profile": Value Change {
        n2101 = event-data() -> ()  [unwired: 1 in, 5 out]
        n2102 = flat-sequence {
          tunnel: w2989 -> [w2992]
          tunnel: w2988 -> [w3000]
          tunnel: [w2994] -> w2987
          tunnel: [w2993] -> w2986
          tunnel: [w2991] -> w2984
          tunnel: [w2990] -> w2981
          tunnel: w2987 -> [w3007]
          tunnel: w2986 -> [w3006]
          tunnel: [w3004] -> w2985
          tunnel: w2984 -> [w3005]
          tunnel: [w3003] -> w2983
          tunnel: [w3002] -> w2982
          tunnel: w2981 -> [w3002]
          tunnel: w2985 -> [w3011]
          tunnel: w2983 -> [w3010]
          tunnel: w2982 -> [w3009]
          frame #0 {
            n2103 = call "Read Stage Position.vi"("error in"=w3000, "VISA resource name in"=w2992) -> ("Current Position"=w2990:cluster{dbl, dbl, dbl}, "error out"=w2993:errorcluster, "VISA resource name out"=w2991:refnum<visa-resource-name>)  [unwired: 1 out]
            "Current Position" <- w2990
            n2104 = local write "Stage Control Serial Error"(w2993) -> ()
            n2105 = Unbundle(w2990) -> (w2997:dbl, w2999:dbl, w2995:dbl)
            n2106 = Add(x=w2999, y="Y change (mm)") -> (x+y=w2996:dbl)
            n2107 = Bundle(w2997, w2996, w2995) -> (w2994:cluster{dbl, dbl, dbl})  [unwired: 1 in]
          }
          frame #1 {
            # "move to new position and start saving"
            n2108 = local write "Stage Moving"(TRUE ("Stage Moving")) -> ()
            n2109 = local write "Start Saving"(TRUE ("Start Saving")) -> ()
            n2110 = call "Set Stage Position.vi"("Position"=w3007, "error in"=w3006, "VISA resource name in"=w3005) -> ("error out"=w3003:errorcluster, "VISA resource name out"=w3004:refnum<visa-resource-name>)  [unwired: 1 out]
          }
          frame #2 {
            # "go back to start"
            n2111 = call "Set Stage Position.vi"("Position"=w3009, "error in"=w3010, "VISA resource name in"=w3011) -> ()  [unwired: 3 out]
          }
          frame #3 {
            # "stop saving"
            n2112 = local write "Stop Saving"(TRUE ("Stop Saving")) -> ()
            n2113 = local write "Stage Moving"(FALSE ("Stage Moving")) -> ()
          }
        }
      }
      event "Move to Position 1", "Move to Position 2", "Move to Position 3", "Move to Position 4", "Move to Position 5", "Lower Ch. Cap.": Value Change {
        n2114 = event-data() -> ()  [unwired: 1 in, 5 out]
        n2115 = Or(x="Move to Position 5", y="Lower Ch. Cap.") -> (x .or. y?=w3020:bool)
        n2116 = Build Array("Move to Position 1", "Move to Position 2", "Move to Position 3", "Move to Position 4", w3020) -> (w3023:bool[])
        n2117 = Boolean Array To Number(Boolean array=w3023) -> (number=w3022:u32)
        n2118 = Logarithm Base 2(1:w3022) -> (0:w3021:dbl)
        n2119 = local write "Move to Position 2"(FALSE ("Move to Position 2")) -> ()
        n2120 = local write "Move to Position 1"(FALSE ("Move to Position 1")) -> ()
        n2121 = flat-sequence {
          tunnel: w3021 -> [w3029]
          tunnel: w3018 -> [w3035]
          tunnel: w3017 -> [w3034]
          tunnel: [w3029] -> w3014
          tunnel: w3014 -> [w3053]
          frame #0 {
            n2122 = local read "Saved Stage Positions"() -> (w3044:dbl[][])
            n2123 = call <vilib>:"Beep.vi"() -> ()  [unwired: 3 in, 9 out]
            n2124 = Array Subset(array=w3044, index (row)=w3029, length (row)=1 ("length"), index (col)=1 ("index"), length (col)=3 ("length")) -> (w3041:dbl[][])
            n2125 = local write "Stage Moving"(TRUE ("Stage Moving")) -> ()
            n2126 = Reshape Array(w3041, 3 ("dimension size")) -> (w3039:dbl[])
            n2127 = Array To Cluster(array=w3039) -> (cluster=w3038:cluster{"[0]":dbl, "[1]":dbl, "[2]":dbl})
            n2128 = property on="Saving Move" class="Bool (strict)"() -> ("Value"=w3031:bool)  [unwired: 2 in, 2 out]
            n2129 = property on="Calibrating..." class="Bool (strict)"() -> ("Value"=w3033:bool)  [unwired: 2 in, 2 out]
            n2130 = Not(x=w3033) -> (.not. x?=w3032:bool)
            n2131 = And(x=w3031, y=w3032) -> (x .and. y?=w3030:bool)
            n2132 = call "Set Stage Position.vi"("Position"=w3038, "error in"=w3034, "VISA resource name in"=w3035) -> ("error out"=w3037:errorcluster)  [unwired: 2 out]
            n2133 = case shown="True" w3030 {
              frame False {
              }
              frame True {
                n2134 = Get Date/Time In Seconds() -> (seconds since 1Jan1904=w3052:timestamp)
                n2135 = Format Date/Time String(time format string (%c)="%H:%M:%S%3u", seconds (now)=w3052, UTC format=TRUE) -> (date/time string=w3049:string)
                n2136 = call <vilib>:"Space Constant.vi"() -> ("String"=w3048:string)
                n2137 = Concatenate Strings(w3049, w3048, "moving") -> (w3046:string)
                n2138 = property on="Move Time" class="Str"("Val(Sgnl)"=w3046) -> ()  [unwired: 2 in, 2 out]
              }
            }
            n2139 = local write "Stage Control Serial Error"(w3037) -> ()
          }
          frame #1 {
            n2140 = call <vilib>:"Beep.vi"() -> ()  [unwired: 3 in, 9 out]
            n2141 = property on="Saving Move" class="Bool (strict)"() -> ("Value"=w3057:bool)  [unwired: 2 in, 2 out]
            n2142 = property on="Calibrating..." class="Bool (strict)"() -> ("Value"=w3055:bool)  [unwired: 2 in, 2 out]
            n2143 = Increment(x=w3053) -> (x+1=w3054:dbl)
            n2144 = Not(x=w3055) -> (.not. x?=w3056:bool)
            n2145 = local write "Stage Moving"(FALSE ("Stage Moving")) -> ()
            n2146 = And(x=w3057, y=w3056) -> (x .and. y?=w3058:bool)
            n2147 = case shown="True" w3058 {
              tunnel: w3054 -> [_ w3060]
              frame False {
              }
              frame True {
                n2148 = Get Date/Time In Seconds() -> (seconds since 1Jan1904=w3068:timestamp)
                n2149 = Format Date/Time String(time format string (%c)="%H:%M:%S%3u", seconds (now)=w3068, UTC format=TRUE) -> (date/time string=w3065:string)
                n2150 = Number To Decimal String(number=w3060, width (-)=1) -> (decimal integer string=w3061:string)
                n2151 = call <vilib>:"Space Constant.vi"() -> ("String"=w3064:string)
                n2152 = Concatenate Strings(w3065, w3064, w3061) -> (w3063:string)
                n2153 = property on="Move Time" class="Str"("Val(Sgnl)"=w3063) -> ()  [unwired: 2 in, 2 out]
              }
            }
          }
        }
      }
      event "Set Current\nPos to 0,0,0": Value Change {
        # "DH is \"Define Home\""
        n2154 = event-data() -> ()  [unwired: 1 in, 6 out]
        n2155 = local write "Set Current\nPos to 0,0,0"(FALSE ("Set Current\nPos to 0,0,0")) -> ()
        n2156 = Concatenate Strings("1DH" ("string"), ";" ("string"), "2DH" ("string"), ";" ("string"), "3DH" ("string"), "\r") -> (w3074:string)
        n2157 = call-poly "VISA Configure Serial Port"("VISA resource name"=w3079, "baud rate (9600)"=u32 19200, "error in (no error)"=w3078) -> ("VISA resource name out"=w3076:refnum<visa-resource-name>, "error out"=w3075:errorcluster)  [unwired: 11 in]
        n2158 = VISA Write(VISA resource name=w3076, write buffer=w3074, error in (no error)=w3075) -> (error out=w3069:errorcluster)  [unwired: 2 out]
        n2159 = local write "Stage Control Serial Error"(w3069) -> ()
      }
      event "Got ADig bead": Value Change {
        n2160 = event-data() -> ()  [unwired: 1 in, 5 out]
        n2161 = flat-sequence {
          frame #0 {
            n2162 = local read "Cap 1 Samp Flow ON"() -> (w3085:bool)
            n2163 = case shown="True" w3085 {
              frame False {
              }
              frame True {
                n2164 = property on="Sample Channel\nFlow" class="Bool (strict)"("Val(Sgnl)"=TRUE ("Value (Signaling)")) -> ()  [unwired: 2 in, 2 out]
              }
            }
            n2165 = local write "Got ADig bead"(FALSE) -> ()
          }
          frame #1 {
            n2166 = property on="Inject Pump 3" class="Bool (strict)"("Val(Sgnl)"=FALSE ("Value (Signaling)")) -> ()  [unwired: 2 in, 2 out]
            n2167 = local write "Target"(FALSE ("Target")) -> ()
          }
          frame #2 {
            n2168 = property on="Move Cap. 1 (DNA Bottom)" class="Bool (strict)"("Val(Sgnl)"=TRUE ("Value (Signaling)")) -> ()  [unwired: 2 in, 2 out]
          }
        }
      }
      event "Force FB Script": Value Change {
        n2169 = event-data() -> ()  [unwired: 1 in, 5 out]
        n2170 = local write "Force FB Script"(FALSE ("Force FB Data\nScript")) -> ()
        n2171 = flat-sequence {
          tunnel: w3096 -> [w3100]
          tunnel: w3097 -> [w3101]
          tunnel: [w3101] -> w3092
          tunnel: [w3100] -> w3091
          tunnel: w3092 -> [w3104]
          tunnel: w3091 -> [w3103]
          tunnel: ["Trap Trig Fl."] -> w3093
          tunnel: [w3146] -> w3094
          tunnel: w3093 -> [w3146]
          tunnel: [w3150] -> w3095
          tunnel: w3094 -> [w3150]
          tunnel: w3095 -> [w3152]
          frame #0 {
            n2172 = property on="Trap D (MHz)" class="DigNum (strict)"("Val(Sgnl)"="Trap D Before Moving") -> ()  [unwired: 2 in, 2 out]
          }
          frame #1 {
            n2173 = local read "Saved Stage Positions"() -> (w3106:dbl[][])
            n2174 = local write "FB Trap Pos Offset"(0.0 ("FB Trap Pos Offset")) -> ()
            n2175 = property on="Trap Pos. FB Offset Factor" class="DigNum (strict)"("Val(Sgnl)"=i64 0 ("Value (Signaling)")) -> ()  [unwired: 2 in, 2 out]
            n2176 = local write "Stage Moving"(TRUE ("Stage Moving")) -> ()
            n2177 = call "move to saved stage position.vi"("error in"=w3103, "Stage VISA resource name in"=w3104, "Position"="Stage Position To Establish FB", "Saved Stage Positions"=w3106) -> ("error out"=w3102:errorcluster)  [unwired: 1 out]
            n2178 = local write "Stage Control Serial Error"(w3102) -> ()
          }
          frame #2 {
            n2179 = call <vilib>:"Beep.vi"("duration (msec)"=u32 100, "frequency (Hz)"=u32 20) -> ()  [unwired: 1 in, 9 out]
            n2180 = local write "Stage Moving"(FALSE ("Stage Moving")) -> ()
            n2181 = property on="Tab Control 2" class="TabCtl (strict)"("Val(Sgnl)"=T6."Feedback on Trap Position" ("Value (Signaling)")) -> ()  [unwired: 2 in, 2 out]
            n2182 = stacked-sequence {
              frame #0 {
                n2183 = Multiply(x="Wait (s)", y=u32 1000 ("milliseconds to wait")) -> (x*y=w3115:u32)
                n2184 = property on="Trap D (MHz)" class="DigNum (strict)"("Val(Sgnl)"="Starting Trap D (MHz)") -> ()  [unwired: 2 in, 2 out]
                n2185 = Wait (ms)(milliseconds to wait=w3115) -> ()  [unwired: 1 out]
              }
              frame #1 {
                n2186 = property on="Set Reading to\nSetpoint" class="Bool (strict)"("Val(Sgnl)"=TRUE ("Value (Signaling)")) -> ()  [unwired: 2 in, 2 out]
              }
            }
            n2187 = property on="Tab Control" class="TabCtl (strict)"("Val(Sgnl)"=T34."Trap Control (RF)" ("Value (Signaling)")) -> ()  [unwired: 2 in, 2 out]
          }